vi "UHR-Fleezers Control (host) - 12.0.vi"() -> ()   [LabVIEW 2014] (continued)
    n3034 = Divide(x=w3759, y=w3760) -> (x/y=→"Sigma/Mean 2":dbl)
    n3035 = Divide(x=w3814, y=w3813) -> (x/y=→"s/Mean":dbl)
    n3036 = feedback-in #26("Calibration") -> ()
    n3037 = feedback #26(u16 1 ("Calibration")) -> (w3843:u16)
    n3038 = Divide(x="T2 offset_x (mV)", y=1000.0) -> (x/y=w3823:dbl)
    n3039 = case shown="0, Default" "Calibration" {
      tunnel: "T1 a_x (nm/V)" -> [_ w4252 w4273]
      tunnel: "T1 k_x (pN/nm)" -> [_ _ w4263]
      tunnel: "T2 a_x (nm/V)" -> [_ w4251 w4271]
      tunnel: "T2 k_x (pN/nm)" -> [_ _ w4264]
      tunnel: w3824 -> [w4234 w4249 w4269]
      tunnel: w3821 -> [w4233 w4247 w4267]
      tunnel: [w4234 w4246 w4266] -> w3852
      tunnel: [w4233 w4245 w4265] -> w3851
      tunnel: ["T1 X (V)" ("Label.Text") "T1 X (nm)" ("Label.Text") "T1 X (pN)" ("Label.Text")] -> w3840
      tunnel: ["T2 X (V)" ("Label.Text") "T2 X (nm)" ("Label.Text") "T2 X (pN)" ("Label.Text")] -> w3839
      tunnel: ["Position (V)" ("Label.Text") "Position (nm)" ("Label.Text") "Force (pN)" ("Label.Text")] -> w3841
      tunnel: w3823 -> [_ w4237 w4256]
      tunnel: w3825 -> [_ w4240 w4258]
      tunnel: ["Mean (V)" ("Label.Text") "Mean (nm)" ("Label.Text") "Mean (pN)" ("Label.Text")] -> w3836
      tunnel: ["Difference (V)" ("Label.Text") "Difference (nm)" ("Label.Text") "Difference (pN)" ("Label.Text")] -> w3778
      frame 0, Default {
      }
      frame 1 {
        n3040 = Unbundle By Name(w4249) -> ("Y"=w4253:dbl[])
        n3041 = Unbundle By Name(w4247) -> ("Y"=w4238:dbl[])
        n3042 = Subtract(x=w4253, y=w4240) -> (x-y=w4241:dbl[])
        n3043 = Subtract(x=w4238, y=w4237) -> (x-y=w4239:dbl[])
        n3044 = Multiply(x=w4239, y=w4251) -> (x*y=w4248:dbl[])
        n3045 = Multiply(x=w4252, y=w4241) -> (x*y=w4250:dbl[])
        n3046 = Bundle By Name(cluster=w4247, "Y"=w4248) -> (w4245:waveform(dbl))
        n3047 = Bundle By Name(cluster=w4249, "Y"=w4250) -> (w4246:waveform(dbl))
      }
      frame 2 {
        n3048 = Unbundle By Name(w4269) -> ("Y"=w4274:dbl[])
        n3049 = Unbundle By Name(w4267) -> ("Y"=w4272:dbl[])
        n3050 = Subtract(x=w4272, y=w4256) -> (x-y=w4257:dbl[])
        n3051 = Subtract(x=w4274, y=w4258) -> (x-y=w4259:dbl[])
        n3052 = Compound Arithmetic op=MULTIPLY(w4257, w4271, w4264) -> (w4268:dbl[])
        n3053 = Compound Arithmetic op=MULTIPLY(w4263, w4273, w4259) -> (w4270:dbl[])
        n3054 = Bundle By Name(cluster=w4267, "Y"=w4268) -> (w4265:waveform(dbl))
        n3055 = Bundle By Name(cluster=w4269, "Y"=w4270) -> (w4266:waveform(dbl))
      }
    }
    n3056 = Not Equal?(x=w3843, y="Calibration") -> (x != y?=w3804:bool)
    n3057 = case shown="True" w3804 {
      tunnel: w3841 -> [_ w4227]
      tunnel: w3840 -> [_ w4226]
      tunnel: w3839 -> [_ w4225]
      tunnel: w3836 -> [_ w4224]
      tunnel: w3778 -> [_ w4223]
      frame False {
      }
      frame True {
        n3058 = property on="Force" class="WFChart (strict)"("YScale.NameLbl.Text"=w4227) -> ()  [unwired: 2 in, 2 out]
        n3059 = property on="T2 X" class="DigNum (strict)"("Caption.Text"=w4225) -> ()  [unwired: 2 in, 2 out]
        n3060 = property on="T1 X" class="DigNum (strict)"("Caption.Text"=w4226) -> ()  [unwired: 2 in, 2 out]
        n3061 = property on="Mean" class="DigNum (strict)"("Caption.Text"=w4224) -> ()  [unwired: 2 in, 2 out]
        n3062 = property on="Difference" class="DigNum (strict)"("Caption.Text"=w4223) -> ()  [unwired: 2 in, 2 out]
      }
    }
    n3063 = Unbundle By Name(w3824) -> ("Y"=w3827:dbl[])
    n3064 = Unbundle By Name(w3821) -> ("Y"=w3830:dbl[])
    n3065 = Subtract(x=w3827, y=w3825) -> (x-y=w3828:dbl[])
    n3066 = Subtract(x=w3830, y=w3823) -> (x-y=w3829:dbl[])
    n3067 = Multiply(x=w3829, y="T2 a_x (nm/V)") -> (x*y=w3631:dbl[])
    n3068 = Multiply(x="T1 a_x (nm/V)", y=w3828) -> (x*y=w3632:dbl[])
    n3069 = Not(x="Trap Trig. Fl.") -> (.not. x?=w3668:bool)
    n3070 = Multiply(x=w3851, y=-1.0) -> (x*y=w3832:waveform(dbl))
    n3071 = Subtract(x=w3632, y=w3631) -> (x-y=w3820:dbl[])
    n3072 = Unbundle By Name(w3851) -> ("Y"=w3794:dbl[])
    n3073 = Unbundle By Name(w3852) -> ("Y"=w3633:dbl[])
    n3074 = Negate(x=w3820) -> (-x=w3629:dbl[])
    n3075 = Build Array(w3852, w3832) -> (→"Force":waveform(dbl)[])
    n3076 = Subtract(x=w3629, y="Offset (nm)") -> (x-y=w3792:dbl[])
    n3077 = case shown="True" "Read Lateness and Rel Phase" {
      tunnel: w3649 -> [w4198 w4222]
      tunnel: w3648 -> [w4199 w4221]
      tunnel: [w4198 w4220] -> w3818
      tunnel: [w4199 w4219] -> w3817
      frame False {
      }
      frame True {
        n3078 = xnode "Read/Write Control"("FPGA VI Reference In"=w4222, "error in"=w4221) -> ("FPGA VI Reference Out"=w4220:T22, "error out"=w4219:errorcluster, "GI Relative phase"=→"GI relative phase":i16, "Relative phase"=→"Relative phase (AI1)":i16, "AI Late Counter"=→"Late Counter (AI1)":u8, "GI Late Counter"=→"GI Late Counter":u8, "MCL Late Counter"=→"MCL Late Counter":u8, "MCL Relative Phase"=→"Relative Phase (MCL)":i16, "APD Acq Relative Phase"=→"APD Acq Relative Phase":i16, "APD 1 Gate Relative Phase"=→"APD 1 Gate Relative Phase":i16, "APD 2 Gate Relative Phase"=→"APD 2 Gate Relative Phase":i16, "APD Acq Late Counter"=→"APD Acq Late Counter":u8, "APD 1 Gate Late Counter"=→"APD 1 Gate Late Counter":u8, "APD 2 Gate Late Counter"=→"APD 2 Gate Late Counter":u8, "Green FB Relative Phase"=→"Relative phase (Green FB)":i16, "GI Relative phase 2"=→"GI relative phase 2":i16, "GI Late Counter 2"=→"GI Late Counter 2":u8, "Trap Pos FIFO Timeout"=→"Trap Pos FIFO Timeout":u16, "Trap AI FIFO Timeout"=→"Trap AI FIFO Timeout":u16, "RI relative phase"=→"RI relative phase":i16, "RI late counter"=→"RI late counter":u8)
      }
    }
    n3079 = call-poly <vilib>:"Mean.vi"("X"=w3794) -> ("mean"=w3635:dbl)  [unwired: 1 out]
    "T2 X" <- w3635
    n3080 = Negate(x=w3794) -> (-x=w3795:dbl[])
    n3081 = call-poly <vilib>:"Mean.vi"("X"=w3633) -> ("mean"=w3636:dbl)  [unwired: 1 out]
    "T1 X" <- w3636
    n3082 = Negate(x=w3635) -> (-x=w3634:dbl)
    n3083 = Bundle By Name(cluster=w3824, "Y"=w3792) -> (w3769:waveform(dbl))
    "Bead Separation" <- w3769
    n3084 = Add(x=w3633, y=w3795) -> (x+y=w3796:dbl[])
    n3085 = Add(x=w3636, y=w3634) -> (x+y=w3838:dbl)
    n3086 = Subtract(x=w3636, y=w3634) -> (x-y=→"Difference":dbl)
    n3087 = Divide(x=w3796, y=2.0) -> (x/y=→"Vec Mean of T1 T2":dbl[])
    n3088 = Divide(x=w3838, y=2.0) -> (x/y=w3798:dbl)
    "Mean" <- w3798
    n3089 = feedback-in #27("Trap Trig. Fl.") -> ()
    n3090 = feedback #27("Trap Trig. Fl.") -> (w3666:bool)
    n3091 = And(x=w3668, y=w3666) -> (x .and. y?=w3667:bool)
    n3092 = case "If have just turned off triggering" shown="True" w3667 {
      tunnel: w3649 -> [_ w4028]
      tunnel: w3648 -> [_ w4027]
      frame False {
      }
      frame True {
        w4026 = FALSE ("FPGA Trap Trig")
        n3093 = xnode "Read/Write Control"("FPGA VI Reference In"=w4028, "error in"=w4027, "FPGA Trap Trig"=w4026) -> ("FPGA VI Reference Out"=w4025:T22, "error out"=w4024:errorcluster)
        n3094 = xnode "Read/Write Control"("FPGA VI Reference In"=w4025, "error in"=w4024, "TTrig?"=w4026) -> ()  [unwired: 2 out]
        n3095 = local write "Initializing"(FALSE ("Initializing")) -> ()
        n3096 = local write "Triggered"(FALSE ("Triggered")) -> ()
        n3097 = local write "Waiting"(FALSE ("Waiting")) -> ()
      }
    }
    n3098 = Not(x=w3666) -> (.not. x?=w3679:bool)
    n3099 = And(x="Trap Trig. Fl.", y=w3679) -> (x .and. y?=w3676:bool)
    n3100 = local read "Tether"() -> (w3799:bool)
    n3101 = Or(x=w3676, y="Reinitialize") -> (x .or. y?=w3662:bool)
    n3102 = feedback #28(w3672) -> (w3677:string)
    n3103 = Select(t=w3672, s=w3676, f=w3677) -> (s? t:f=w3671:string)
    n3104 = Select(t=w3672, s="Reinitialize", f=w3671) -> (s? t:f=w3670:string)
    n3105 = feedback #29(0) -> (w3674:i32)
    n3106 = feedback #30(w3792) -> (w3791:dbl[])
    n3107 = Build Array (concatenate)(w3792, w3791) -> (w3630:dbl[])
    n3108 = case "For determining if there is a tether still" shown="True" w3799 {
      tunnel: w3798 -> [_ w4152]
      frame False {
      }
      frame True {
        n3109 = Greater?(x="Lost Tether Alarm Threshold (pN)", y=w4152) -> (0:w4150:bool)
        n3110 = case shown="True" w4150 {
          frame False {
          }
          frame True {
            w4153 = TRUE
            w4157 = FALSE ("Multiple tether")
            w4158 = FALSE ("Value (Signaling)")
            n3111 = flat-sequence {
              frame #0 {
                # "stop only if saving"
                n3112 = local read "Saving..."() -> (w4170:bool)
                n3113 = And(x=w4170, y="TA Cancel Save?") -> (x .and. y?=w4169:bool)
                n3114 = local write "Stop Saving"(w4169) -> ()
              }
              frame #1 {
                n3115 = case shown="True" "TA Green Off?" {
                  frame False {
                  }
                  frame True {
                    w4173 = FALSE ("Fl. Triggered...")
                    n3116 = local write "Fl. Triggered..."(w4173) -> ()
                    n3117 = property on="Green ON/Interlacing" class="Bool (strict)"("Val(Sgnl)"=w4173) -> ()  [unwired: 2 in, 2 out]
                  }
                }
              }
            }
            n3118 = local read "Time tether formed"() -> (w4164:timestamp)
            n3119 = Get Date/Time In Seconds() -> (seconds since 1Jan1904=w4165:timestamp)
            n3120 = Subtract(x=w4165, y=w4164) -> (x-y=w4163:dbl)
            n3121 = Number To Decimal String(number=w4163) -> (decimal integer string=w4160:string)  [unwired: 1 out]
            n3122 = local read "Messages"() -> (w4167:string)
            n3123 = call <vilib>:"Beep.vi"("use system alert? (T)"=FALSE, "duration (msec)"=u32 200, "frequency (Hz)"=u32 200) -> ()  [unwired: 9 out]
            n3124 = Concatenate Strings("Lost tether (" ("Message to add"), w4160, " s)." ("string")) -> (w4162:string)
            n3125 = local write "Tether"(FALSE ("Tether")) -> ()
            n3126 = call "Update messages.vi"("Message to add"=w4162, "Old message string"=w4167) -> ("New message string"=w4166:string)
            n3127 = local write "Messages"(w4166) -> ()
            n3128 = local write "Pause dwell"(w4158) -> ()
            n3129 = property on="Fl. Triggered..." class="Bool (strict)"("Val(Sgnl)"=w4158) -> ()  [unwired: 2 in, 2 out]
            n3130 = local write "Dip for Protein"(w4158) -> ()
            n3131 = property on="Trap Pos. FB ON" class="Bool (strict)"("Val(Sgnl)"=w4158) -> ()  [unwired: 2 in, 2 out]
            n3132 = property on="Trap Trig. Fl." class="Bool (strict)"("Val(Sgnl)"=w4158) -> ()  [unwired: 2 in, 2 out]
            n3133 = local write "Multiple tether"(w4157) -> ()
            n3134 = local write "Bad fit"(w4157) -> ()
            n3135 = local write "Hysteresis"(w4157) -> ()
            n3136 = local write "Good tether"(w4157) -> ()
            n3137 = local write "Save scans"(w4153) -> ()
            n3138 = local write "Restart DMA? (AOD)"(w4153) -> ()
          }
        }
      }
    }
    n3139 = case "For triggering actions based on the trap position (e.g., turning the excitation laser on if trap under feedback moves so far)" shown="True" "Trap Trig. Fl." {
      tunnel: w3657 -> [_ w4041]
      tunnel: w3670 -> [_ w4040]
      tunnel: ["" ("t") w4039] -> w3678
      tunnel: w3662 -> [_ w4038]
      tunnel: [0 ("t") w4037] -> w3675
      tunnel: w3674 -> [_ w4036]
      tunnel: w3649 -> [_ w4035]
      tunnel: w3648 -> [_ w4034]
      frame False {
      }
      frame True {
        n3140 = case shown="\"Wait for trigger\"" w4040 {
          tunnel: w4041 -> [w4058 _ _ w4106]
          tunnel: [w4055 w4087 "" ("t") w4109] -> w4039
          tunnel: w4038 -> [_ _ _ w4097]
          tunnel: [w4054 w4084 0 ("t") w4098] -> w4037
          tunnel: w4036 -> [_ w4086 _ w4104]
          tunnel: w4035 -> [w4043 w4081 _ w4100]
          tunnel: w4034 -> [w4042 w4080 _ w4099]
          frame "Wait for trigger" {
            n3141 = local read "Trap Trig. (FPGA)"() -> (w4046:bool)
            n3142 = Subtract(x=w4058, y="Mean T1 Position\nto compare (nm)") -> (x-y=w4051:dbl[])
            n3143 = call <vilib>:"Std Deviation and Variance.vi"("X"=w4051) -> ("mean"=→"mean":dbl, "standard deviation"=→"standard\ndeviation":dbl)  [unwired: 1 in, 1 out]
            n3144 = Array Max & Min(array=w4051) -> (max value=→"max value":dbl, min value=→"min value":dbl)  [unwired: 2 out]
            n3145 = Greater?(x=w4051, y="Threshold (nm)") -> (0:w4061:bool[])
            n3146 = case shown="True" w4046 {
              tunnel: w4043 -> [_ w4067]
              tunnel: w4042 -> [_ w4066]
              tunnel: [FALSE ("TTrig?") w4065] -> w4049
              frame False {
              }
              frame True {
                n3147 = xnode "Read/Write Control"("FPGA VI Reference In"=w4067, "error in"=w4066) -> ("TTrig?"=w4065:bool)  [unwired: 2 out]
              }
            }
            n3148 = Or Array Elements(Boolean array=w4061) -> (logical OR=w4048:bool)
            n3149 = Select(t=w4049, s=w4046, f=w4048) -> (s? t:f=w4047:bool)
            n3150 = Not(x=w4046) -> (.not. x?=w4045:bool)
            n3151 = And(x=w4047, y=w4045) -> (x .and. y?=w4044:bool)
            n3152 = Select(t="Triggered", s=w4047, f="Wait for trigger") -> (s? t:f=w4055:string)
            n3153 = case shown="True" w4047 {
              tunnel: [0 0] -> w4054
              tunnel: w4043 -> [_ w4072]
              tunnel: w4042 -> [_ w4071]
              frame False {
                "Waiting" <- TRUE ("Waiting")
              }
              frame True {
                n3154 = xnode "Read/Write Control"("FPGA VI Reference In"=w4072, "error in"=w4071, "TTrig?"=FALSE) -> ()  [unwired: 2 out]
                n3155 = local read "Messages"() -> (w4075:string)
                n3156 = call <vilib>:"Beep.vi"() -> ()  [unwired: 12 in]
                n3157 = call "Update messages.vi"("Message to add"="Unwinding trigger.", "Old message string"=w4075) -> ("New message string"=w4076:string)
                n3158 = local write "Messages"(w4076) -> ()
                n3159 = local write "Waiting"(FALSE ("Waiting")) -> ()
                "Triggered" <- TRUE ("Triggered")
              }
            }
            n3160 = case "Only need to turn on laser if host triggered" shown="True" w4044 {
              frame False {
              }
              frame True {
                n3161 = property on="Green ON/Interlacing" class="Bool (strict)"("Val(Sgnl)"=TRUE ("Value (Signaling)")) -> ()  [unwired: 2 in, 2 out]
              }
            }
          }
          frame "Triggered" {
            n3162 = local read "Trap Trig. (FPGA)"() -> (w4083:bool)
            n3163 = Increment(x=w4086) -> (x+1=w4084:i32)
            n3164 = Greater Or Equal?(x=w4084, y="Fl. ON time (n)") -> (x >= y?=w4082:bool)
            n3165 = Select(t="Wait for trigger", s=w4082, f="Triggered" ("t")) -> (s? t:f=w4087:string)
            n3166 = And(x=w4082, y=w4083) -> (x .and. y?=w4079:bool)
            n3167 = case shown="True" w4079 {
              tunnel: w4081 -> [_ w4091]
              tunnel: w4080 -> [_ w4090]
              frame False {
              }
              frame True {
                n3168 = xnode "Read/Write Control"("FPGA VI Reference In"=w4091, "error in"=w4090, "FPGA Trap Trig"=TRUE) -> ()  [unwired: 2 out]
              }
            }
            n3169 = case shown="True" w4082 {
              frame False {
              }
              frame True {
                w4093 = FALSE ("Value (Signaling)")
                n3170 = local write "Triggered"(w4093) -> ()
                n3171 = local write "Waiting"(TRUE ("Waiting")) -> ()
                n3172 = property on="Green ON/Interlacing" class="Bool (strict)"("Val(Sgnl)"=w4093) -> ()  [unwired: 2 in, 2 out]
              }
            }
          }
          frame "Do nothing" {
          }
          frame "Initialize", Default {
            n3173 = Increment(x=w4104) -> (x+1=w4108:i32)
            n3174 = Select(t=1, s=w4097, f=w4108) -> (s? t:f=w4098:i32)
            n3175 = feedback #31(w4106) -> (w4112:dbl[])
            n3176 = Build Array (concatenate)(w4106, w4112) -> (w4105:dbl[])
            n3177 = Greater Or Equal?(x=w4098, y="Wait to get offset (n)") -> (x >= y?=w4101:bool)
            n3178 = Select(t=w4106, s=w4097, f=w4105) -> (s? t:f=w4107:dbl[])
            n3179 = feedback-in #31(w4107) -> ()
            n3180 = call-poly <vilib>:"Mean.vi"("X"=w4107) -> ("mean"=w4102:dbl)  [unwired: 1 out]
            n3181 = local write "Mean T1 Position\nto compare (nm)"(w4102) -> ()
            n3182 = case shown="True" w4097 {
              tunnel: w4100 -> [_ w4118]
              tunnel: w4099 -> [_ w4117]
              frame False {
              }
              frame True {
                w4114 = FALSE ("FPGA Trap Trig")
                n3183 = xnode "Read/Write Control"("FPGA VI Reference In"=w4118, "error in"=w4117, "FPGA Trap Trig"=w4114) -> ("FPGA VI Reference Out"=w4116:T22, "error out"=w4115:errorcluster)
                n3184 = xnode "Read/Write Control"("FPGA VI Reference In"=w4116, "error in"=w4115, "TTrig?"=w4114) -> ()  [unwired: 2 out]
              }
            }
            n3185 = Select(t="Wait for trigger", s=w4101, f="Initialize") -> (s? t:f=w4109:string)
            n3186 = case shown="True" w4101 {
              tunnel: w4102 -> [_ w4121]
              tunnel: w4100 -> [_ w4130]
              tunnel: w4099 -> [_ w4129]
              frame False {
                n3187 = local write "Waiting"(FALSE ("Waiting")) -> ()
                "Initializing" <- TRUE ("Initializing")
              }
              frame True {
                n3188 = local read "Threshold (nm)"() -> (w4133:dbl)
                n3189 = local read "AOM X Cal (nm/MHz)"() -> (w4132:dbl)
                n3190 = Add(x=w4121, y=w4133) -> (x+y=w4134:dbl)
                n3191 = Divide(x=w4134, y=w4132) -> (x/y=w4131:dbl)
                n3192 = call "IR AOM freq to word.vi"("Frequency In (MHz)"=w4131) -> ("Frequency Word Out (double)"=w4128:dbl)
                n3193 = local write "Initializing"(FALSE ("Initializing")) -> ()
                n3194 = local write "Waiting"(TRUE ("Waiting")) -> ()
                n3195 = To Quad Integer(1:w4128) -> (0:w4127:i64)
                n3196 = xnode "Read/Write Control"("FPGA VI Reference In"=w4130, "error in"=w4129, "FPGA TTrig Thresh"=w4127) -> ("FPGA VI Reference Out"=w4124:T22, "error out"=w4123:errorcluster)
                n3197 = xnode "Read/Write Control"("FPGA VI Reference In"=w4124, "error in"=w4123, "FPGA Trap Trig"=TRUE) -> ()  [unwired: 2 out]
              }
            }
          }
        }
      }
    }
    n3198 = feedback-in #28(w3678) -> ()
    n3199 = feedback-in #29(w3675) -> ()
    n3200 = Split 1D Array(array=w3630, index=w3692) -> (first subarray=w3788:dbl[])  [unwired: 1 out]
    n3201 = feedback-in #30(w3788) -> ()
    n3202 = call-poly <vilib>:"Mean.vi"("X"=w3788) -> ("mean"=w3787:dbl)  [unwired: 1 out]
    "Bead Mean (nm)" <- w3787
    n3203 = Subtract(x=w3788, y=w3787) -> (x-y=w3786:dbl[])
    n3204 = Square(x=w3786) -> (x^2=w3785:dbl[])
    n3205 = call-poly <vilib>:"Mean.vi"("X"=w3785) -> ("mean"=w3784:dbl)  [unwired: 1 out]
    n3206 = Square Root(x=w3784) -> (sqrt(x)=w3783:dbl)
    n3207 = Multiply(x=10.0, y=w3783) -> (x*y=→"RMS (Å)":dbl)
    n3208 = xnode ("Read/Write Control")("FPGA VI Reference In"=w3818, "error in"=w3817) -> ("FPGA VI Reference Out"=w3660:T22, "error out"=w3659:errorcluster, "AI2 Y Sum Set 1"=w3913:i16, "AI2 Y Sum Set 2"=w3912:i16, "AI1 X Set 1"=w3720:fxp<+/-,16,1>, "AI1 X Set 2"=w3719:fxp<+/-,16,1>, "Trap Pos FB Int Signal"=→"Trap Pos FB Int Signal":fxp<+/-,24,9>, "Trap Pos FB Int-Norm Signal"=→"Trap Pos FB Int-Norm Signal":fxp<+/-,16,1>, "Trap Pos FB Action"=w3713:i64, "Scanning"=→"AOD Scanning":bool, "Scan I"=→"AOD Scan I":u64, "Scanning MCL"=w3915:bool, "Scan I (MCL)"=→"MCL Scan I":u64, "Green FB Sum"=w3855:i16, "Trap Pos FB Action"=w3647:i64, "Wiggling 1"=→"Wiggling T1":bool, "TTrig Fin Thresh"=w3643:i64, "Wiggling 2"=→"Wiggling T2":bool, "Red FB Sum"=w3610:i16)  [unwired: 2 out]
    "MCL Scanning" <- w3915
    "Trap Pos FB Action" <- w3713
    n3209 = local read "FB Trig Integrate"() -> (w3641:u32)
    n3210 = Divide(x=w3855, y=3276.7) -> (x/y=w3609:dbl)
    "Green laser intensity (V)" <- w3609
    n3211 = Divide(x=w3610, y=3276.7) -> (x/y=w3608:dbl)
    "Red laser intensity (V)" <- w3608
    n3212 = Divide(x=w3647, y=w3641) -> (x/y=w3640:dbl)
    "TTrig Sig (Int)" <- w3640
    n3213 = Divide(x=w3643, y=w3641) -> (x/y=w3638:dbl)
    "TTrig Fin Thresh (Int)" <- w3638
    n3214 = local read "AOM X Cal (nm/MHz)"() -> (w3646:dbl)
    n3215 = local read "AI2 (V)"() -> (w3914:cluster{"Set 1":dbl, "Set 2":dbl})
    n3216 = Bundle By Name(cluster=w3914, "Set 1"=w3913, "Set 2"=w3912) -> (w3910:cluster{"Set 1":dbl, "Set 2":dbl})
    n3217 = Divide(x=w3713, y=327.67) -> (x/y=w3625:dbl)
    n3218 = local read "Trap X (AI1)"() -> (w3733:T10)
    n3219 = Bundle(w3609, w3608) -> (→"Excitation laser intensities plot":cluster{dbl, dbl})  [unwired: 1 in]
    n3220 = call "IR AOM word double to freq.vi"("Frequency Word In (double)"=w3638) -> ("Frequency Out (MHz)"=w3637:dbl)
    n3221 = call "IR AOM word double to freq.vi"("Frequency Word In (double)"=w3640) -> ("Frequency Out (MHz)"=w3639:dbl)
    n3222 = Divide(x=w3910, y=3276.7) -> (x/y=w3909:cluster{"Set 1":dbl, "Set 2":dbl})
    n3223 = Multiply(x=w3639, y=w3646) -> (x*y=w3645:dbl)
    "TTrig Sig (nm)" <- w3645
    n3224 = Multiply(x=w3637, y=w3646) -> (x*y=w3644:dbl)
    "TTrig Fin Thresh (nm)" <- w3644
    n3225 = local write "AI2 (V)"(w3909) -> ()
    n3226 = local read "Trap Pos. FB Range"() -> (w3624:T12)
    n3227 = Bundle(cluster=w3733, "Trap 1"=w3720, "Trap 2"=w3719) -> (→"Trap X (AI1)":T10)
    n3228 = Bundle(w3645, w3644) -> (→"TTrig":cluster{dbl, dbl})  [unwired: 1 in]
    n3229 = Unbundle(w3624) -> ("output high"=w3623:fxp<+/-,64,32>)  [unwired: 1 out]
    n3230 = Divide(x=w3625, y=w3623) -> (x/y=→"Action (%)":dbl)
    n3231 = flat-sequence "To save data" {
      tunnel: [w4994] -> w3932
      tunnel: [w4995] -> w3931
      tunnel: w3885 -> [w4967]
      tunnel: w3665 -> [w4992]
      tunnel: ["Save Calibration"] -> w3906
      tunnel: w3903 -> [w4991]
      tunnel: [w4985] -> w3902
      tunnel: [w4982] -> w3901
      tunnel: [w4979] -> w3900
      tunnel: w3884 -> [w4981]
      tunnel: w3802 -> [w4975]
      tunnel: [w4975] -> w3801
      tunnel: ["Start Saving"] -> w3771
      tunnel: [w4969] -> w3705
      tunnel: [w4968] -> w3704
      tunnel: w3932 -> [w5234]
      tunnel: w3931 -> [w5233]
      tunnel: w3706 -> [w5232]
      tunnel: w3906 -> [w5231]
      tunnel: w3902 -> [w5229]
      tunnel: w3901 -> [w5228]
      tunnel: w3900 -> [w5227]
      tunnel: w3780 -> [w5226]
      tunnel: w3811 -> [w5225]
      tunnel: w3801 -> [w5224]
      tunnel: w3771 -> [w5223]
      tunnel: w3769 -> [w5222]
      tunnel: w3747 -> [w5221]
      tunnel: w3705 -> [w5220]
      tunnel: w3704 -> [w5219]
      tunnel: w3703 -> [w5218]
      tunnel: w3626 -> [w5217]
      frame #0 {
        n3232 = Or(x="Save N Sets", y="Start Saving") -> (x .or. y?=w4976:bool)
        n3233 = To Double Precision Float(number=w4991) -> (double precision float=w4986:dbl)
        n3234 = Build Array(w4976, "Save Calibration", w4967, w4981) -> (w4990:bool[])
        n3235 = Compound Arithmetic op=OR("Save Calibration", w4967, w4976, w4981) -> (w4993:bool)
        n3236 = Boolean Array To Number(Boolean array=w4990) -> (number=w4988:u32)
        n3237 = feedback #32(FALSE ("Save APD Data\nwith Trap Data")) -> (w4970:bool)
        n3238 = feedback #33(refnum<k0> refnum) -> (w4996:refnum<file>)
        n3239 = feedback #34(refnum<k0> refnum) -> (w4972:refnum<file>)
        n3240 = feedback #35(FALSE ("Save APD Data\nwith Trap Data")) -> (w4980:bool)
        n3241 = feedback #36(refnum<k0> refnum) -> (w4983:refnum<file>)
        n3242 = feedback #37(0) -> (w4998:i32)
        n3243 = feedback #38() -> (w4987:u32)  [unwired: 1 out]
        n3244 = case shown="True" w4993 {
          tunnel: [w5005 1] -> w4994
          tunnel: w4998 -> [w5007 _]
          tunnel: [w5006 w5025] -> w4995
          tunnel: w4996 -> [w5006 _]
          tunnel: w4992 -> [_ w5045]
          tunnel: w4986 -> [_ w5043]
          tunnel: w4988 -> [_ w5046]
          tunnel: [w5004 w5024] -> w4985
          tunnel: w4987 -> [w5004 _]
          tunnel: [w5003 w5022] -> w4982
          tunnel: w4983 -> [w5003 _]
          tunnel: [w5002 w5021] -> w4979
          tunnel: w4980 -> [w5002 _]
          tunnel: "Start Saving" -> [_ w5019]
          tunnel: w4975 -> [_ w5018]
          tunnel: [w5001 w5009] -> w4968
          tunnel: w4972 -> [w5001 _]
          tunnel: [w5000 w5008] -> w4969
          tunnel: w4970 -> [w5000 _]
          frame False {
            n3245 = Increment(x=w5007) -> (x+1=w5005:i32)
          }
          frame True {
            w5015 = FALSE ("Start Saving")
            w5020 = 9.0  # File Version
            w5028 = FALSE ("prepend array or string size? (T)")
            w5026 = T29."big-endian, network order" ("byte order (0:big-endian, network order)")
            n3246 = local read "BD 1 Frequency 1 (MHz)"() -> (w5042:dbl)
            n3247 = local read "BD 2 Frequency 1 (MHz)"() -> (w5041:dbl)
            n3248 = local read "BD 1 Frequency 2 (MHz)"() -> (w5040:dbl)
            n3249 = local read "BD 2 Frequency 2 (MHz)"() -> (w5039:dbl)
            n3250 = local read "BD 1 Frequency 3 (MHz)"() -> (w5038:dbl)
            n3251 = local read "BD 2 Frequency 3 (MHz)"() -> (w5037:dbl)
            n3252 = Array Size(array=w5018) -> (size(s)=w5017:i32)
            n3253 = To Double Precision Float(number=w5017) -> (double precision float=w5016:dbl)
            n3254 = local write "Save Calibration"(w5015) -> ()
            n3255 = local write "Start Saving"(w5015) -> ()
            n3256 = Build Array("Save APD Data\nwith Trap Data", "Save Trap Pos. Data") -> (w5012:bool[])
            n3257 = Boolean Array To Number(Boolean array=w5012) -> (number=w5011:u32)
            n3258 = Build Array(w5042, w5041, w5040, w5039, w5038, w5037) -> (w5036:dbl[])
            n3259 = case shown="1, Default" w5046 {
              tunnel: w5045 -> [w5119 w5141 w5157 w5195]
              tunnel: w5016 -> [w5124 w5148 w5177 w5214]
              tunnel: w5043 -> [w5123 w5147 w5176 w5213]
              tunnel: [w5120 w5143 w5168 w5205] -> w5034
              tunnel: [w5112 "Cal sets to save" w5158 w5196] -> w5024
              tunnel: w5036 -> [w5121 w5144 w5170 w5207]
              tunnel: "Save APD Data\nwith Trap Data" -> [w5118 _ w5154 w5193]
              tunnel: [w5118 FALSE ("Save APD Data\nwith Trap Data") w5154 w5193] -> w5021
              tunnel: w5020 -> [w5115 w5138 w5152 w5191]
              tunnel: w5019 -> [w5114 _ _ _]
              tunnel: [w5106 "Active cal?" w5151 w5181] -> w5008
              tunnel: "Save Trap Pos. Data" -> [w5106 _ w5151 w5181]
              tunnel: w5011 -> [w5105 _ w5150 w5180]
              frame 1, Default {
                # "timeseries"
                n3260 = case shown="True" "Profile" {
                  tunnel: [w5127 w5131] -> w5110
                  tunnel: [w5127 w5130] -> w5109
                  tunnel: [w5127 w5129] -> w5108
                  tunnel: [w5127 w5128] -> w5107
                  frame False {
                    w5127 = 0.0 ("f")
                  }
                  frame True {
                    n3261 = local read "Current Position"() -> (w5132:cluster{dbl, dbl, dbl})
                    n3262 = local read "Y change (mm)"() -> (w5128:dbl)
                    n3263 = Unbundle(w5132) -> (w5131:dbl, w5130:dbl, w5129:dbl)
                  }
                }
                n3264 = local read "Save ave N"() -> (w5126:dbl)
                n3265 = Multiply(x=w5126, y=w5119) -> (x*y=w5125:dbl)
                n3266 = To Double Precision Float(number=w5105) -> (double precision float=w5117:dbl)
                n3267 = Select(t=4.0, s="Profile", f=0.0) -> (s? t:f=w5101:dbl)
                n3268 = Build Array(w5115, w5119, w5125, w5124, w5123, w5101) -> (w5122:dbl[])
                n3269 = Build Array(w5117, w5110, w5109, w5108, w5107) -> (w5116:dbl[])
                n3270 = Select(t=u32 4000000000, s=w5114, f="N sets to save") -> (s? t:f=w5112:u32)
                n3271 = Build Array (concatenate)(w5122, w5121, w5116) -> (w5120:dbl[])
              }
              frame 2 {
                w5140 = 0.0 ("f")
                # "If doing active calibration,\nalso save trap position file"
                # "calibration"
                n3272 = property on="Wiggle" class="Bool (strict)"("Val(Sgnl)"="Active cal?") -> ()  [unwired: 2 in, 2 out]
                n3273 = Select(t=2.0, s="Active cal?", f=0.0) -> (s? t:f=w5134:dbl)
                n3274 = Build Array(w5134, w5140, w5140, w5140, w5140) -> (w5139:dbl[])
                n3275 = Build Array(w5138, w5141, w5141, w5148, w5147, 1.0 ("t")) -> (w5145:dbl[])
                n3276 = Build Array (concatenate)(w5145, w5144, w5139) -> (w5143:dbl[])
                "Calibrating..." <- TRUE ("Calibrating...")
              }
              frame 4 {
                w5155 = 0.0 ("f")
                # "scan dir (x/y = 0/1)"
                # "cycles/step"
                # "n scans (f/b)"
                # "steps"
                # "freq. range"
                # "AOD raster scan"
                n3277 = local read "Number of F/B Scans (AOD)"() -> (w5162:u16)
                n3278 = local read "Cycles/step (AOD)"() -> (w5164:u64)
                n3279 = local read "Scan Range (MHz)"() -> (w5167:dbl)
                n3280 = local read "Scan steps (AOD)"() -> (w5166:u64)
                n3281 = local read "Scan BD"() -> (w5174:bool)
                n3282 = local read "Save ave N"() -> (w5179:dbl)
                n3283 = Boolean To (0,1)(Boolean=w5174) -> (0, 1=w5173:i16)
                n3284 = To Double Precision Float(number=w5162) -> (double precision float=w5161:dbl)
                n3285 = To Double Precision Float(number=w5166) -> (double precision float=w5165:dbl)
                n3286 = To Double Precision Float(number=w5164) -> (double precision float=w5163:dbl)
                n3287 = To Double Precision Float(number=w5173) -> (double precision float=w5172:dbl)
                n3288 = Multiply(x=w5179, y=w5157) -> (x*y=w5178:dbl)
                n3289 = To Double Precision Float(number=w5150) -> (double precision float=w5156:dbl)
                n3290 = Build Array(w5156, w5155, w5155, w5155, w5155) -> (w5153:dbl[])
                n3291 = local read "N sets should be saved"() -> (w5159:dbl)
                n3292 = Build Array(w5172, w5167, w5165, w5163, w5161) -> (w5169:dbl[])
                n3293 = Build Array(w5152, w5157, w5178, w5177, w5176, 2.0 ("t")) -> (w5171:dbl[])
                n3294 = Round Toward +Infinity(x=w5159) -> (ceil(x): smallest int >= x=w5160:dbl)
                n3295 = Build Array (concatenate)(w5171, w5170, w5153, w5169) -> (w5168:dbl[])
                n3296 = To Unsigned Long Integer(number=w5160) -> (unsigned 32bit integer=w5158:u32)
              }
              frame 8 {
                w5188 = 0.0 ("f")
                # "MCL raster scan"
                n3297 = local read "Number of scans (MCL)"() -> (w5183:u64)
                n3298 = local read "Scan lines (y)"() -> (w5182:u64)
                n3299 = local read "2D or 1D Scan"() -> (w5185:bool)
                n3300 = local read "Scan Range (V)\n(of steps)"() -> (w5204:dbl)
                n3301 = local read "Fast Scan Dir"() -> (w5211:bool)
                n3302 = local read "Cycles/step (MCL)"() -> (w5201:u64)
                n3303 = local read "Scan steps (MCL)"() -> (w5203:u64)
                n3304 = Select(t=w5182, s=w5185, f=w5183) -> (s? t:f=w5184:u64)
                n3305 = Boolean To (0,1)(Boolean=w5185) -> (0, 1=w5187:i16)
                n3306 = local read "Save ave N"() -> (w5216:dbl)
                n3307 = local read "Initial X"() -> (w5190:dbl)
                n3308 = local read "Initial Y"() -> (w5189:dbl)
                n3309 = To Double Precision Float(number=w5187) -> (double precision float=w5186:dbl)
                n3310 = Boolean To (0,1)(Boolean=w5211) -> (0, 1=w5210:i16)
                n3311 = To Double Precision Float(number=w5184) -> (double precision float=w5199:dbl)
                n3312 = To Double Precision Float(number=w5203) -> (double precision float=w5202:dbl)
                n3313 = To Double Precision Float(number=w5201) -> (double precision float=w5200:dbl)
                n3314 = To Double Precision Float(number=w5210) -> (double precision float=w5209:dbl)
                n3315 = Multiply(x=w5216, y=w5195) -> (x*y=w5215:dbl)
                n3316 = To Double Precision Float(number=w5180) -> (double precision float=w5194:dbl)
                n3317 = local read "N sets should be saved (MCL)"() -> (w5197:dbl)
                n3318 = Build Array(w5194, w5186, w5188, w5188, w5188) -> (w5192:dbl[])
                n3319 = Build Array(w5209, w5204, w5202, w5200, w5199, w5190, w5189) -> (w5206:dbl[])
                n3320 = Build Array(w5191, w5195, w5215, w5214, w5213, 3.0 ("t")) -> (w5208:dbl[])
                n3321 = Round Toward +Infinity(x=w5197) -> (ceil(x): smallest int >= x=w5198:dbl)
                n3322 = Build Array (concatenate)(w5208, w5207, w5192, w5206) -> (w5205:dbl[])
                n3323 = To Unsigned Long Integer(number=w5198) -> (unsigned 32bit integer=w5196:u32)
              }
            }
            n3324 = local read "Index"() -> (w5051:dbl)
            n3325 = call "Create new save file.vi"("Insert"="", "Ext"=".dat", "Index In"=w5051) -> ("Path Out"=w5010:path, "Index Out"=w5023:dbl)
            n3326 = local write "Save file name"(w5010) -> ()
            n3327 = local write "Index"(w5023) -> ()
            n3328 = local write "Save index"(w5023) -> ()
            n3329 = Array Size(array=w5034) -> (size(s)=w5035:i32)
            n3330 = Open/Create/Replace File(file path (use dialog)=w5010, operation (0:open)=T30."create", access (0:read/write)=enum16{"read/write", "read-only", "write-only"}."write-only") -> (refnum out=w5048:refnum<file>)  [unwired: 1 in, 4 out]
            n3331 = local write "Saving..."(TRUE ("Saving...")) -> ()
            n3332 = To Double Precision Float(number=w5035) -> (double precision float=w5033:dbl)
            n3333 = String Length(string="Comment (data description)") -> (length=w5031:i32)
            n3334 = To Double Precision Float(number=w5031) -> (double precision float=w5030:dbl)
            n3335 = Deny Access(7:w5048) -> (3:w5047:refnum<file>)  [unwired: 1 in, 2 out]
            n3336 = Build Array (concatenate)(w5033, w5034, w5030) -> (w5032:dbl[])
            n3337 = case "If fluorescence data to be saved" shown="True" w5021 {
              tunnel: w5010 -> [_ w5100]
              tunnel: [refnum<k0> refnum w5080] -> w5022
              frame False {
              }
              frame True {
                w5079 = 0.0
                n3338 = local read "APD Integration Time (s)"() -> (w5085:dbl)
                n3339 = local read "N APD Samp/step"() -> (w5078:dbl)
                n3340 = Path To String(path=w5100) -> (string=w5099:string)
                n3341 = String Length(string=w5099) -> (length=w5098:i32)
                n3342 = Subtract(x=w5098, y=4) -> (x-y=w5096:i32)
                n3343 = String Subset(string=w5099, length (rest)=w5096) -> (substring=w5095:string)  [unwired: 1 out]
                n3344 = Build Array(w5085, w5078, w5079, w5079, w5079, w5079, w5079, w5079) -> (w5082:dbl[])
                n3345 = Concatenate Strings(w5095, "_fl.dat" ("string")) -> (w5093:string)
                n3346 = Array Size(array=w5082) -> (size(s)=w5084:i32)
                n3347 = String To Path(string=w5093) -> (path=w5089:path)
                n3348 = Open/Create/Replace File(file path (use dialog)=w5089, operation (0:open)=T30."create", access (0:read/write)=enum16{"read/write", "read-only", "write-only"}."write-only") -> (refnum out=w5090:refnum<file>)  [unwired: 1 in, 4 out]
                n3349 = Deny Access(7:w5090) -> (3:w5086:refnum<file>)  [unwired: 1 in, 2 out]
                n3350 = To Double Precision Float(number=w5084) -> (double precision float=w5083:dbl)
                n3351 = Build Array (concatenate)(w5083, w5082) -> (w5081:dbl[])
                n3352 = Write to Binary File(file (use dialog)=w5086, data=w5081, 5:FALSE ("prepend array or string size? (T)"), 9:T29."big-endian, network order" ("byte order (0:big-endian, network order)")) -> (refnum out=w5080:refnum<file>)  [unwired: 1 in, 3 out]
              }
            }
            n3353 = case shown="True" w5008 {
              tunnel: w5010 -> [_ w5062]
              tunnel: [refnum<k0> refnum w5061] -> w5009
              frame False {
              }
              frame True {
                w5057 = 0.0 ("element")
                n3354 = Path To String(path=w5062) -> (string=w5076:string)
                n3355 = Build Array(w5057, w5057, w5057, w5057, w5057, w5057, w5057, w5057) -> (w5058:dbl[])
                n3356 = String Length(string=w5076) -> (length=w5075:i32)
                n3357 = Subtract(x=w5075, y=4) -> (x-y=w5073:i32)
                n3358 = Array Size(array=w5058) -> (size(s)=w5060:i32)
                n3359 = String Subset(string=w5076, length (rest)=w5073) -> (substring=w5072:string)  [unwired: 1 out]
                n3360 = To Double Precision Float(number=w5060) -> (double precision float=w5059:dbl)
                n3361 = Concatenate Strings(w5072, "_pos.dat" ("string")) -> (w5070:string)
                n3362 = Build Array (concatenate)(w5059, w5058) -> (w5056:dbl[])
                n3363 = String To Path(string=w5070) -> (path=w5066:path)
                n3364 = Open/Create/Replace File(file path (use dialog)=w5066, operation (0:open)=T30."create", access (0:read/write)=enum16{"read/write", "read-only", "write-only"}."write-only") -> (refnum out=w5067:refnum<file>)  [unwired: 1 in, 4 out]
                n3365 = Deny Access(7:w5067) -> (3:w5063:refnum<file>)  [unwired: 1 in, 2 out]
                n3366 = Write to Binary File(file (use dialog)=w5063, data=w5056, 5:FALSE ("prepend array or string size? (T)"), 9:T29."big-endian, network order" ("byte order (0:big-endian, network order)")) -> (refnum out=w5061:refnum<file>)  [unwired: 1 in, 3 out]
              }
            }
            n3367 = Write to Binary File(file (use dialog)=w5047, data=w5032, 5:w5028, 9:w5026) -> (refnum out=w5029:refnum<file>)  [unwired: 1 in, 3 out]
            n3368 = Write to Binary File(file (use dialog)=w5029, data="Comment (data description)", 5:w5028, 9:w5026) -> (refnum out=w5025:refnum<file>)  [unwired: 1 in, 3 out]
          }
        }
        n3369 = feedback-in #32(w4969) -> ()
        n3370 = feedback-in #33(w4995) -> ()
        n3371 = feedback-in #34(w4968) -> ()
        n3372 = feedback-in #35(w4979) -> ()
        n3373 = feedback-in #36(w4982) -> ()
        n3374 = feedback-in #37(w4994) -> ()
        n3375 = feedback-in #38(w4985) -> ()
      }
      frame #1 {
        n3376 = local read "Saving..."() -> (w5230:bool)
        n3377 = case shown="True" w5230 {
          tunnel: w5234 -> [_ w5246]
          tunnel: w5233 -> [_ w5259]
          tunnel: w5232 -> [_ w5255]
          tunnel: w5231 -> [_ w5254]
          tunnel: w5229 -> [_ w5235]
          tunnel: w5228 -> [_ w5249]
          tunnel: w5227 -> [_ w5248]
          tunnel: w5226 -> [_ w5247]
          tunnel: w5225 -> [_ w5245]
          tunnel: w5224 -> [_ w5243]
          tunnel: w5223 -> [_ w5242]
          tunnel: w5222 -> [_ w5241]
          tunnel: w5221 -> [_ w5240]
          tunnel: w5220 -> [_ w5239]
          tunnel: w5219 -> [_ w5238]
          tunnel: w5218 -> [_ w5237]
          tunnel: w5217 -> [_ w5236]
          frame False {
          }
          frame True {
            n3378 = Multiply(x=w5246, y=w5245) -> (x*y=→"Time (s)":dbl)
            n3379 = Less Or Equal?(x=w5246, y=w5235) -> (x <= y?=w5257:bool)
            n3380 = Or(x="Stop Saving", y="Abort save 2") -> (x .or. y?=w5250:bool)
            n3381 = Not(x=w5250) -> (.not. x?=w5258:bool)
            n3382 = And(x=w5257, y=w5258) -> (x .and. y?=w5256:bool)
            n3383 = case shown="True" w5256 {
              tunnel: w5259 -> [w5267 w5342]
              tunnel: [0.0 w5345] -> w5253
              tunnel: w5246 -> [_ w5343]
              tunnel: w5235 -> [_ w5344]
              tunnel: w5255 -> [_ w5339]
              tunnel: w5254 -> [_ _]
              tunnel: w5249 -> [w5265 w5332]
              tunnel: w5248 -> [w5264 w5333]
              tunnel: w5247 -> [_ w5331]
              tunnel: w5243 -> [_ w5330]
              tunnel: w5242 -> [_ w5274]
              tunnel: w5241 -> [_ w5323]
              tunnel: w5240 -> [_ w5301]
              tunnel: w5239 -> [w5261 w5283]
              tunnel: w5238 -> [w5262 w5282]
              tunnel: w5237 -> [_ w5279]
              tunnel: w5236 -> [_ w5277]
              frame False {
                w5263 = FALSE
                n3384 = Close File(refnum=w5267) -> ()  [unwired: 1 in, 2 out]
                n3385 = case shown="True" w5264 {
                  tunnel: w5265 -> [_ w5269]
                  frame False {
                  }
                  frame True {
                    n3386 = Close File(refnum=w5269) -> ()  [unwired: 1 in, 2 out]
                  }
                }
                n3387 = case shown="True" w5261 {
                  tunnel: w5262 -> [_ w5268]
                  frame False {
                  }
                  frame True {
                    n3388 = Close File(refnum=w5268) -> ()  [unwired: 1 in, 2 out]
                  }
                }
                n3389 = call <vilib>:"Beep.vi"() -> ()  [unwired: 3 in, 9 out]
                n3390 = local write "Raster Scanning..."(w5263) -> ()
                n3391 = local write "Calibrating..."(w5263) -> ()
                n3392 = property on="Abort wiggle" class="Bool (strict)"("Val(Sgnl)"=TRUE) -> ()  [unwired: 2 in, 2 out]
                n3393 = local write "Stop Saving"(w5263) -> ()
                "Saving..." <- w5263
              }
              frame True {
                n3394 = local read "Calibrating..."() -> (w5334:bool)
                n3395 = case "Write fl. data" shown="True" w5333 {
                  tunnel: w5332 -> [_ w5368]
                  tunnel: w5331 -> [_ w5367]
                  frame False {
                  }
                  frame True {
                    n3396 = Write to Binary File(file (use dialog)=w5368, data=w5367, 5:FALSE ("prepend array or string size? (T)"), 9:T29."big-endian, network order" ("byte order (0:big-endian, network order)")) -> ()  [unwired: 1 in, 4 out]
                  }
                }
                n3397 = Greater?(x="Save ave N", y=1.0) -> (0:w5337:bool)
                n3398 = Not(x=w5334) -> (.not. x?=w5336:bool)
                n3399 = And(x=w5336, y=w5337) -> (x .and. y?=w5280:bool)
                n3400 = case shown="True" w5280 {
                  tunnel: w5279 -> [w5348 w5359]
                  tunnel: [w5348 w5351] -> w5278
                  tunnel: "Save ave N" -> [_ w5352]
                  frame False {
                  }
                  frame True {
                    w5349 = 2 ("dimension size")
                    n3401 = Array Size(array=w5359) -> (size(s)=w5353:i32)
                    n3402 = Divide(x=w5353, y=w5349) -> (x/y=w5357:dbl)
                    n3403 = Reshape Array(w5359, w5357, w5349) -> (w5358:u64[][])
                    n3404 = Transpose 2D Array(2D array=w5358) -> (transposed array=w5356:u64[][])
                    n3405 = for {
                      tunnel: w5356 -> [w5361] mode=indexing
                      tunnel: [w5360] -> w5350 mode=indexing
                      tunnel: w5352 -> [w5362]
                      workers-P: _ -> [_]
                      n3406 = call "downsample 1D array - U64.vi"("Ave N"=w5362, "Array In"=w5361) -> ("Array Out"=w5360:u64[])  [unwired: 1 in]
                    }
                    n3407 = Transpose 2D Array(2D array=w5350) -> (transposed array=w5355:u64[][])
                    n3408 = Divide(x=w5353, y=w5352) -> (x/y=w5354:dbl)
                    n3409 = Reshape Array(w5355, w5354) -> (w5351:u64[])
                  }
                }
                n3410 = case shown="True" w5280 {
                  tunnel: w5339 -> [w5371 w5383]
                  tunnel: [w5371 w5375] -> w5335
                  tunnel: "Save ave N" -> [_ w5376]
                  tunnel: w5330 -> [_ w5374]
                  frame False {
                  }
                  frame True {
                    n3411 = Array Size(array=w5383) -> (size(s)=w5377:i32)
                    n3412 = Array Size(array=w5374) -> (size(s)=w5373:i32)
                    n3413 = Divide(x=w5377, y=w5373) -> (x/y=w5381:dbl)
                    n3414 = Reshape Array(w5383, w5381, w5373) -> (w5382:i16[][])
                    n3415 = Transpose 2D Array(2D array=w5382) -> (transposed array=w5380:i16[][])
                    n3416 = for {
                      tunnel: w5380 -> [w5386] mode=indexing
                      tunnel: [w5385] -> w5372 mode=indexing
                      tunnel: w5376 -> [w5384]
                      workers-P: _ -> [_]
                      n3417 = call "downsample 1D array - I16.vi"("Ave N"=w5384, "Array In"=w5386) -> ("Array Out"=w5385:i16[])  [unwired: 1 out]
                    }
                    n3418 = Transpose 2D Array(2D array=w5372) -> (transposed array=w5379:i16[][])
                    n3419 = Divide(x=w5377, y=w5376) -> (x/y=w5378:dbl)
                    n3420 = Reshape Array(w5379, w5378) -> (w5375:i16[])
                  }
                }
                n3421 = Index Array(array=w5301, index=1) -> (element=w5304:waveform(dbl))
                n3422 = Index Array(array=w5301, index=0) -> (element=w5306:waveform(dbl))
                n3423 = Unbundle By Name(w5304) -> ("Y"=w5308:dbl[])
                n3424 = Unbundle By Name(w5306) -> ("Y"=w5316:dbl[])
                n3425 = case "Write trap pos. data" shown="True" w5283 {
                  tunnel: w5282 -> [_ w5364]
                  tunnel: w5278 -> [_ w5363]
                  frame False {
                  }
                  frame True {
                    n3426 = Write to Binary File(file (use dialog)=w5364, data=w5363, 5:FALSE ("prepend array or string size? (T)"), 9:T29."big-endian, network order" ("byte order (0:big-endian, network order)")) -> ()  [unwired: 1 in, 4 out]
                  }
                }
                n3427 = Write to Binary File(file (use dialog)=w5342, data=w5335, 5:FALSE ("prepend array or string size? (T)"), 9:T29."big-endian, network order" ("byte order (0:big-endian, network order)")) -> ()  [unwired: 1 in, 4 out]
                n3428 = feedback #39(w5308) -> (w5310:dbl[])
                n3429 = Build Array (concatenate)(w5310, w5308) -> (w5309:dbl[])
                n3430 = Select(t=w5308, s=w5274, f=w5309) -> (s? t:f=w5294:dbl[])
                n3431 = feedback-in #39(w5294) -> ()
                n3432 = feedback #40(w5316) -> (w5329:dbl[])
                n3433 = Build Array (concatenate)(w5329, w5316) -> (w5328:dbl[])
                n3434 = Select(t=w5316, s=w5274, f=w5328) -> (s? t:f=w5303:dbl[])
                n3435 = feedback-in #40(w5303) -> ()
                n3436 = Divide(x=w5343, y=w5344) -> (x/y=w5346:dbl)
                n3437 = Multiply(x=w5346, y=100.0) -> (x*y=w5345:dbl)
                n3438 = Build Array(w5303, w5294) -> (→"Saved APD":dbl[][])
                n3439 = Array Size(array=w5303) -> (size(s)=w5321:i32)
                n3440 = Unbundle By Name(w5323) -> ("Y"=w5327:dbl[])
                n3441 = Subtract(x=w5321, y="N pts to average") -> (x-y=w5297:i32)
                n3442 = Multiply(x="N pts to average", y=u16 2) -> (x*y=w5298:u16)
                n3443 = Subtract(x=w5321, y=w5298) -> (x-y=w5296:i32)
                n3444 = feedback #41(w5327) -> (w5326:dbl[])
                n3445 = Build Array (concatenate)(w5326, w5327) -> (w5325:dbl[])
                n3446 = Select(t=w5327, s=w5274, f=w5325) -> (s? t:f=w5324:dbl[])
                "Trap Delta Graph" <- w5324
                n3447 = feedback-in #41(w5324) -> ()
                n3448 = Array Subset(array=w5303, index=w5297, length="N pts to average") -> (w5320:dbl[])
                n3449 = Array Subset(array=w5303, index=w5296, length="N pts to average") -> (w5319:dbl[])
                n3450 = Array Subset(array=w5294, index=w5297, length="N pts to average") -> (w5300:dbl[])
                n3451 = Array Subset(array=w5294, index=w5296, length="N pts to average") -> (w5299:dbl[])
                n3452 = Index Array(array=w5277, index=0) -> (element=w5275:waveform(dbl))
                n3453 = call-poly <vilib>:"Mean.vi"("X"=w5320) -> ("mean"=w5318:dbl)  [unwired: 1 out]
                n3454 = call-poly <vilib>:"Mean.vi"("X"=w5300) -> ("mean"=w5293:dbl)  [unwired: 1 out]
                n3455 = call-poly <vilib>:"Mean.vi"("X"=w5319) -> ("mean"=w5317:dbl)  [unwired: 1 out]
                n3456 = call-poly <vilib>:"Mean.vi"("X"=w5299) -> ("mean"=w5292:dbl)  [unwired: 1 out]
                n3457 = Unbundle By Name(w5275) -> ("Y"=w5272:dbl[])
                n3458 = Subtract(x=w5293, y=w5292) -> (x-y=w5284:dbl)
                "Delta Fl. 2" <- w5284
                n3459 = Subtract(x=w5318, y=w5317) -> (x-y=w5315:dbl)
                "Delta Fl. 1" <- w5315
                n3460 = Initialize Array(w5315, 1 ("dimension size")) -> (w5312:dbl[])
                n3461 = Initialize Array(w5284, 1 ("dimension size")) -> (w5289:dbl[])
                n3462 = feedback #42(w5312) -> (w5313:dbl[])
                n3463 = Build Array (concatenate)(w5313, w5312) -> (w5311:dbl[])
                n3464 = feedback #43(w5289) -> (w5290:dbl[])
                n3465 = Build Array (concatenate)(w5290, w5289) -> (w5288:dbl[])
                n3466 = feedback #44(w5272) -> (w5271:dbl[])
                n3467 = Build Array (concatenate)(w5271, w5272) -> (w5273:dbl[])
                n3468 = Select(t=w5272, s=w5274, f=w5273) -> (s? t:f=w5270:dbl[])
                "Saved trap pos" <- w5270
                n3469 = feedback-in #44(w5270) -> ()
                n3470 = Select(t=w5312, s=w5274, f=w5311) -> (s? t:f=w5287:dbl[])
                n3471 = feedback-in #42(w5287) -> ()
                n3472 = Select(t=w5289, s=w5274, f=w5288) -> (s? t:f=w5286:dbl[])
                n3473 = feedback-in #43(w5286) -> ()
                n3474 = Build Array(w5287, w5286) -> (→"Save APD Deriv":dbl[][])
              }
            }
            "Progress" <- w5253
            "Progress 2" <- w5253
          }
        }
      }
    }
    n3475 = local read "wait to reset values"() -> (w3917:bool)
    n3476 = Not(x=w3915) -> (.not. x?=w3918:bool)
    n3477 = And(x=w3918, y=w3917) -> (x .and. y?=w3919:bool)
    n3478 = case "Part of MCL raster scanning: returns to initial positions after scan done" shown="True" w3919 {
      tunnel: w3660 -> [w4788 w4795]
      tunnel: [w4788 w4794] -> w3921
      tunnel: w3659 -> [w4787 w4793]
      tunnel: [w4787 w4792] -> w3916
      frame False {
      }
      frame True {
        w4803 = 10.0 ("y")
        w4802 = 32767.0 ("y")
        # "to return scan values\nafter a synchronous \nAOM scan"
        n3479 = local read "AO2"() -> (w4796:dbl)
        n3480 = local read "AO1"() -> (w4797:dbl)
        n3481 = local write "wait to reset values"(FALSE ("wait to reset values")) -> ()
        n3482 = Multiply(x=w4797, y=w4802) -> (x*y=w4799:dbl)
        n3483 = Multiply(x=w4796, y=w4802) -> (x*y=w4801:dbl)
        n3484 = Divide(x=w4799, y=w4803) -> (x/y=w4798:dbl)
        n3485 = Divide(x=w4801, y=w4803) -> (x/y=w4800:dbl)
        n3486 = To Word Integer(number=w4798) -> (16bit integer=w4804:i16)
        n3487 = To Word Integer(number=w4800) -> (16bit integer=w4805:i16)
        n3488 = local read "Total Counts (ticks)"() -> (w4789:u32)
        n3489 = xnode "Read/Write Control"("FPGA VI Reference In"=w4795, "error in"=w4793, "AO1"=w4804, "AO2"=w4805, "MCL count"=w4789) -> ("FPGA VI Reference Out"=w4794:T22, "error out"=w4792:errorcluster)
        n3490 = local read "Scan Range (V)\n(of steps)"() -> (w4790:dbl)
        n3491 = property on="Scan Range (V)\n(of steps)" class="DigNum (strict)"("Val(Sgnl)"=w4790) -> ()  [unwired: 2 in, 2 out]
      }
    }
    n3492 = node-c288() -> ()  [unwired: 2 out]
  }
  n3493 = VISA Close(VISA resource name=w129, error in (no error)=w128) -> (error out=w172:errorcluster)
  n3494 = call <vilib>:"Simple Error Handler.vi"("error in (no error)"=w172) -> ()  [unwired: 1 in, 8 out]
  n3495 = node-c288(w134) -> ()  [unwired: 1 out]
  n3496 = node-c288(w216) -> ()  [unwired: 1 out]
  n3497 = flat-sequence {
    tunnel: w307 -> [w5390]
    tunnel: w309 -> [w5391]
    tunnel: [w5389] -> w289
    tunnel: [w5388] -> w288
    tunnel: w272 -> [_]
    tunnel: w224 -> [_]
    tunnel: w140 -> [_]
    tunnel: w289 -> [w5392]
    tunnel: w288 -> [w5393]
    frame #0 {
      w5387 = FALSE ("AI to FIFO")
      n3498 = xnode "Read/Write Control"("FPGA VI Reference In"=w5391, "error in"=w5390, "AI to FIFO"=w5387, "APD to FIFO"=w5387) -> ("FPGA VI Reference Out"=w5389:T22, "error out"=w5388:errorcluster)
    }
    frame #1 {
      n3499 = xnode "Close FPGA VI Reference"("FPGA VI Reference In"=w5392, "error in"=w5393) -> ("error out"=→"error out":errorcluster)
    }
  }
